vi "Main.vi"() -> ()   [LabVIEW 2020] (continued)
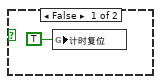
[diagram p2: hidden frame]
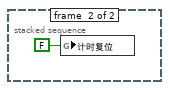
[diagram p3: hidden frame]
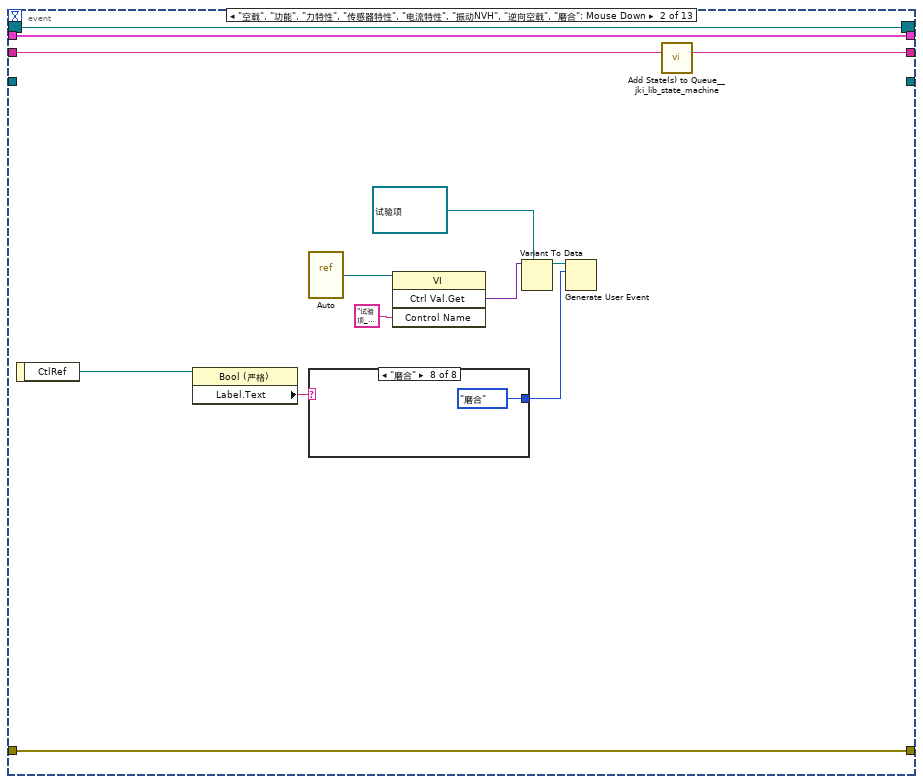
[diagram p4: hidden frame]
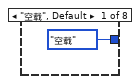
[diagram p5: hidden frame]
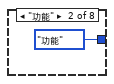
[diagram p6: hidden frame]
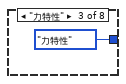
[diagram p7: hidden frame]
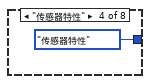
[diagram p8: hidden frame]
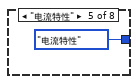
[diagram p9: hidden frame]
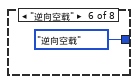
[diagram p10: hidden frame]
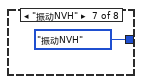
[diagram p11: hidden frame]
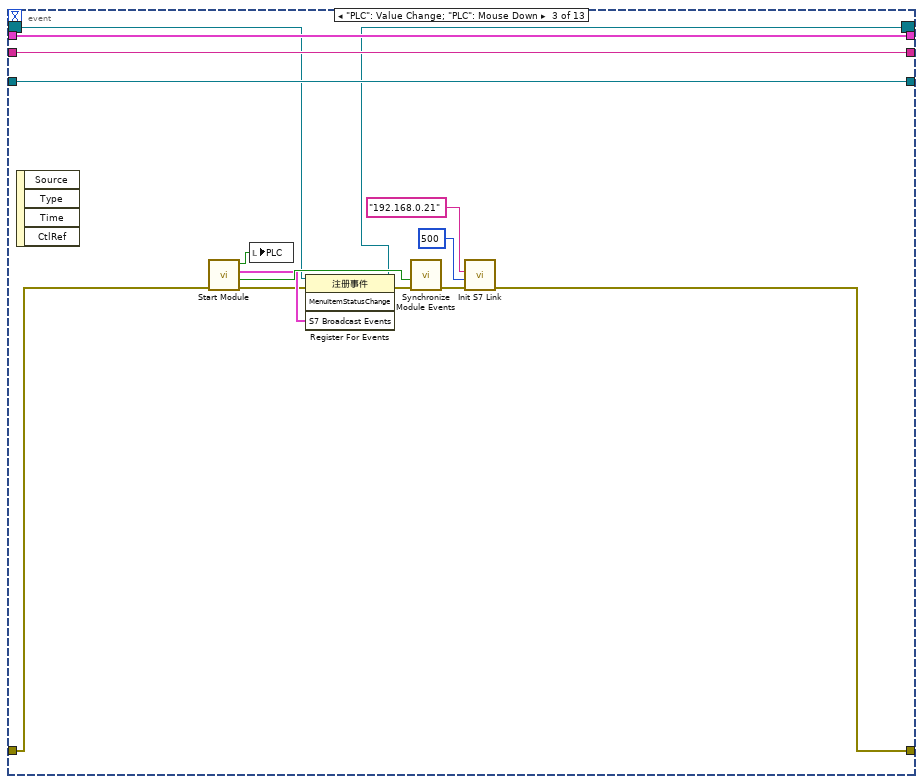
[diagram p12: hidden frame]
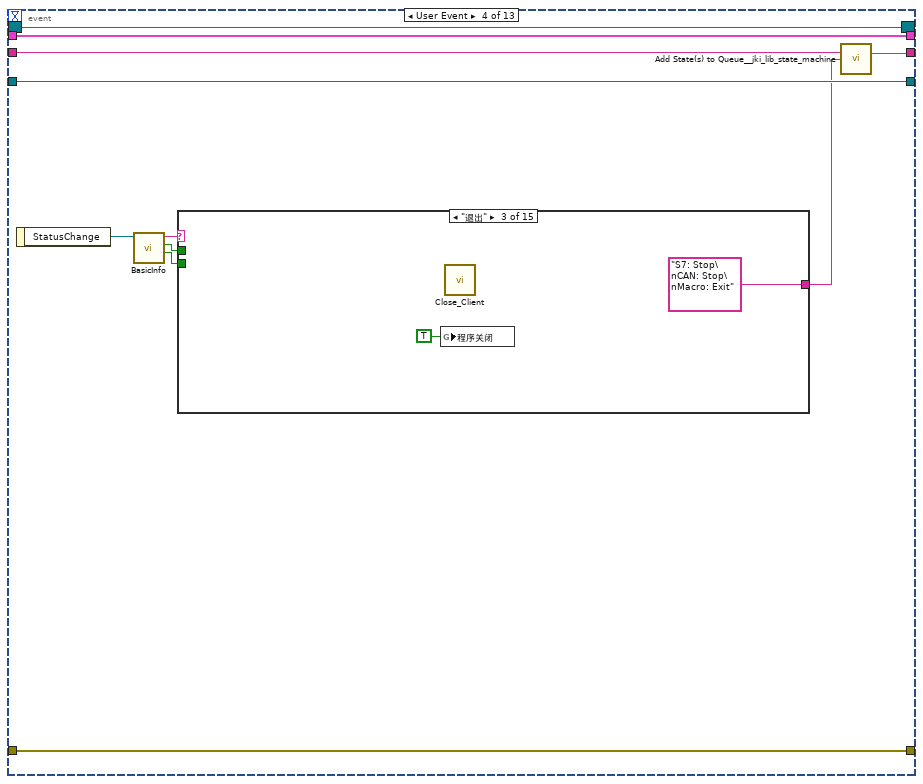
[diagram p13: hidden frame]
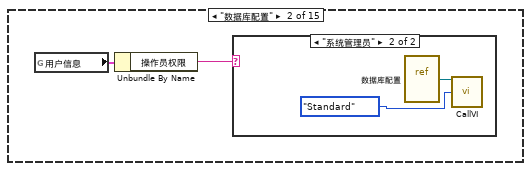
[diagram p15: hidden frame]
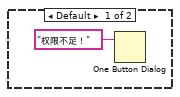
[diagram p16: hidden frame]
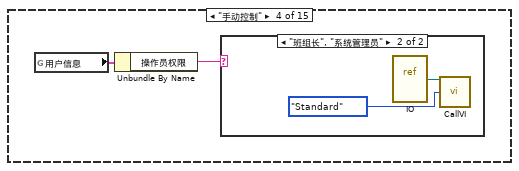
[diagram p17: hidden frame]
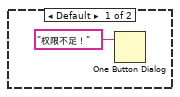
[diagram p18: hidden frame]
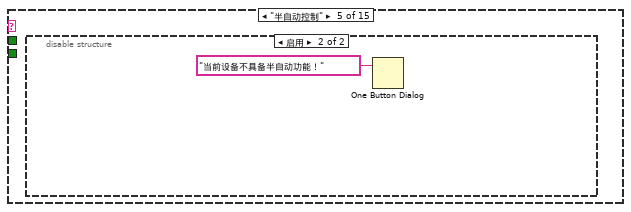
[diagram p19: hidden frame]
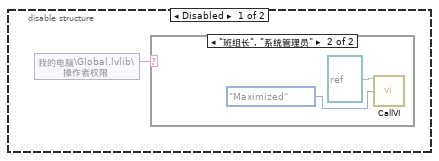
[diagram p20: hidden frame]
                n119 = case shown="真" w200 {
                  frame False {
                  }
                  frame True {
                    n120 = vi-ref "Auto.vi"() -> (w204:refnum<vi>)
                    n121 = invoke class="VI" method="Ctrl Val.Set"(reference=w204, "Control Name"="STEP" ("控件名"), "Value"="退出自动" ("控件名")) -> ()  [unwired: 2 in, 5 out]
                  }
                }
              }
            }
            n122 = call <vilib>:"Add State(s) to Queue__jki_lib_state_machine.vi"("State(s) in (\"\")"=w191) -> ("States Out"=w192:string)  [unwired: 14 in]
          }
          event "错误": Mouse Down {
            n123 = event-data() -> ()  [unwired: 1 in, 8 out]
            n124 = vi-ref "报警信息.vi"() -> (w207:refnum<vi>)
            n125 = call "CallVI.vi"("VI引用"=w207, "状态"=T3."Standard") -> ()  [unwired: 12 in, 2 out]
            n126 = call <vilib>:"Add State(s) to Queue__jki_lib_state_machine.vi"("State(s) in (\"\")"=w209) -> ("States Out"=w210:string)  [unwired: 14 in]
          }
          event Panel Close? {
            n127 = event-data() -> ()  [unwired: 1 in, 1 out]
            n128 = call "Close.vi"() -> ()  [unwired: 11 in, 1 out]
            n129 = global write "Global.vi" "程序关闭"(TRUE ("程序关闭")) -> ()
            n130 = call <vilib>:"Add State(s) to Queue__jki_lib_state_machine.vi"("State(s) in Front (\"\")"="S7: Stop\nMacro: Exit", "State(s) in (\"\")"=w219) -> ("States Out"=w218:string)  [unwired: 13 in]
            n131 = event-data("Discard?"=TRUE) -> ()  [unwired: 1 in, 1 out]
          }
          event "更换产品": Value Change {
            n132 = event-data() -> ("NewVal"=w222:refnum<vi>)  [unwired: 1 in, 5 out]
            n133 = stacked-sequence {
              tunnel: w222 -> [w228]
              tunnel: [w227] -> w220
              frame #0 {
                n134 = stacked-sequence {
                  tunnel: w228 -> [w236 _ _]
                  tunnel: [_ w239 _] -> w227
                  frame #0 {
                    n135 = disable-structure shown="禁用" {
                      disable-tunnel: w236 -> [w238 _]
                      frame Disabled {
                        n136 = control-ref of="子面板"() -> (w237:refnum<vi>)
                        n137 = call "Call_SubPanal.vi"("VI引用句柄"=w238, "SubPnl引用句柄"=w237) -> ()  [unwired: 9 in, 1 out]
                      }
                      frame Enabled {
                      }
                    }
                    n138 = vi-ref "Auto.vi"() -> (w235:refnum<vi>)
                    n139 = invoke class="VI" method="Ctrl Val.Get"(reference=w235, "Control Name"="产品变更_Event" ("控件名")) -> ("Get Control Value Variant"=w233:variant)  [unwired: 2 in, 3 out]
                    n140 = global read "Global.vi" "产品型号"() -> (w230:string)
                    n141 = Variant To Data(type=refnum<user-event> refnum ("产品变更_Event"), Variant=w233) -> (data=w231:refnum<user-event>, error out=w229:errorcluster)  [unwired: 1 in]
                    n142 = Generate User Event(user event=w231, event data cluster=w230, error in=w229) -> ()  [unwired: 1 in, 2 out]
                    n143 = local write "产品型号"(w230) -> ()
                  }
                  frame #1 {
                    n144 = global read "Global.vi" "启用CAN"() -> (w240:bool)
                    n145 = case shown="真" w240 {
                      tunnel: ["CAN: Stop" "CAN: Stop\nIdle\nCAN: Start"] -> w239
                      frame False {
                      }
                      frame True {
                      }
                    }
                  }
                  frame #2 {
                    n146 = control-ref of="磨合"() -> (w243:refnum<vi>)
                    n147 = control-ref of="空载"() -> (w248:refnum<vi>)
                    n148 = control-ref of="功能"() -> (w249:refnum<vi>)
                    n149 = control-ref of="力特性"() -> (w250:refnum<vi>)
                    n150 = control-ref of="电流特性"() -> (w247:refnum<vi>)
                    n151 = control-ref of="传感器特性"() -> (w246:refnum<vi>)
                    n152 = control-ref of="逆向空载"() -> (w245:refnum<vi>)
                    n153 = control-ref of="振动NVH"() -> (w244:refnum<vi>)
                    n154 = global read "Global.vi" "试验项目"() -> (w253:bool[])
                    n155 = Build Array(w248, w249, w250, w247, w246, w245, w244, w243) -> (w252:refnum<vi>[])
                    n156 = for {
                      tunnel: w252 -> [w257] mode=indexing
                      tunnel: w253 -> [w258] mode=indexing
                      shift-right: [w254] -> _
                      shift-left: 2095 -> [w255]
                      i -> [w256]
                      n157 = case shown="真" w258 {
                        tunnel: w257 -> [w259 w267]
                        tunnel: w256 -> [_ _]
                        tunnel: w255 -> [w261 w264]
                        tunnel: [w261 w262] -> w254
                        frame False {
                          n158 = property class="Bool (严格)"(reference=w259, "Top"=2000) -> ()  [unwired: 1 in, 2 out]
                        }
                        frame True {
                          n159 = Add(x=w264, y=115) -> (x+y=w262:i32)
                          n160 = Bundle(w262, 1300) -> (w265:cluster{i32, i32})  [unwired: 1 in]
                          n161 = property class="Bool (严格)"(reference=w267, "Position"=w265) -> ()  [unwired: 1 in, 2 out]
                        }
                      }
                    }
                  }
                }
              }
            }
            n162 = call <vilib>:"Add State(s) to Queue__jki_lib_state_machine.vi"("State(s) in Front (\"\")"=w220, "State(s) in (\"\")"=w223) -> ("States Out"=w224:string)  [unwired: 13 in]
          }
          event "Andon": Value Change {
            n163 = event-data() -> ("NewVal"=w272:enum32{"未选择", "缺料报警", "质量报警", "故障报警"})  [unwired: 1 in]
            n164 = case shown="\"未选择\", 默认" w272 {
              tunnel: [enum16{"设备离线", "设备正常", "设备缺料", "设备故障", "质量报警"}."设备正常" ("设备状态") enum16{"设备离线", "设备正常", "设备缺料", "设备故障", "质量报警"}."设备缺料" ("设备状态") enum16{"设备离线", "设备正常", "设备缺料", "设备故障", "质量报警"}."质量报警" ("设备状态") enum16{"设备离线", "设备正常", "设备缺料", "设备故障", "质量报警"}."设备故障" ("设备状态")] -> w270
              frame "未选择", Default {
              }
              frame "缺料报警" {
              }
              frame "质量报警" {
              }
              frame "故障报警" {
              }
            }
            n165 = local read "userName"() -> (w269:string)
            n166 = Bundle By Name(cluster=T4 {"设备名称"="最终性能试验台1", "操作人员"="", "设备状态"=enum."设备离线", "附加信息"=""} ("设备信息"), "操作人员"=w269, "设备状态"=w270) -> (w268:T4)
            n167 = call "Change_Client.vi"("设备信息"=w268) -> ()  [unwired: 10 in, 1 out]
          }
        }
      }
      frame "---------- Core ----------" {
        n168 = call <vilib>:"Add State(s) to Queue__jki_lib_state_machine.vi"("State(s) in (\"\")"=w286) -> ("States Out"=w285:string)  [unwired: 14 in]
      }
      frame Default {
        w298 = 42 items=["No error", "Argument error", "Memory is full", "Out of zone", "End of file", "File already open", "Generic file I/O error", "File not found", "File permission error", "Disk is full", "Duplicate path", "Too many files open", "System feature not enabled", "Resource file not found", "Cannot add resource", "Resource not found", "Image not found", "Image memory error", "Pen does not exist", "Config type invalid", "Config token not found", "Config parse error", "Config memory error", "Bad external code format", "Bad external code offset", "External code not present", "Null window", "Destroy window error", "Null menu", "Print aborted", "Bad print record", "Print driver error", "Windows error during printing", "Memory error during printing", "Print dialog error", "Generic print error", "Invalid device refnum", "Device not found", "Device parameter error", "Device unit error", "Cannot open device", "Device call aborted", "Generic error", "Cancelled by user", "Object ID too low", "Object ID too high", "Object not in heap", "Unknown heap", "Unknown object (invalid DefProc)", "Unknown object (DefProc not in table)", "Message out of range", "Invalid (null) method", "Unknown message", "Manager call not supported", "Bad address", "Network operation in progress", "Network operation timed out", "Connection is busy", "Network attribute not supported", "Network error", "Address in use", "System out of memory", "Connection aborted", "Connection refused", "Not connected", "Already connected", "Connection closed", "Initialization error (interapplication manager)", "Bad occurrence", "Wait on unbound occurrence handler", "Occurrence queue overflow", "Datalog type conflict", "Unused", "Unrecognized type (interapplication manager)", "Memory corrupt", "Failed to make temporary DLL", "Old CIN version", "Drag socket not found", "Failed to load drop-object", "Failed to register OLE object", "Failed to release OLE object", "Format specifier type mismatch", "Unknown format specifier", "Too few format specifiers", "Too many format specifiers", "Scan failed", "Newer CIN version", "Error converting to variant", "Runtime menu error", "Password tampered", "Variant attribute not found", "Incompatible variant data type", "Event data is not available", "Event Store is not present", "Occurrence is not found", "Event Queue is not created", "Event info is not available", "Refnum passed is NULL", "Error retrieving Class GUID", "Error retrieving CoClass GUID", "Error retrieving TypeLib GUID.", "Bad built application magic bytes.", "Specific driver is different from the specific driver associated with the Logical Name.", "There is no session opened to the class driver.", "Max Error", "MAX - Error with config objects", "MAX - Error loading configuration", "MAX - Group not supported"]
        # "Current State"
        n169 = Format Into String(format string="Software Exception: Unhandled State \"%s\"." ("message"), error in=w294, w289) -> (resulting string=w297:string, error out=w296:errorcluster)  [unwired: 1 in]
        n170 = call <vilib>:"Error Cluster From Error Code.vi"("show call chain? (False)"=TRUE, "error in (no error)"=w296, "error message (\"\")"=w297, "error code (0)"=w298) -> ("error out"=w295:errorcluster)  [unwired: 5 in]
        n171 = call <vilib>:"Add State(s) to Queue__jki_lib_state_machine.vi"("State(s) in (\"\")"=w293) -> ("States Out"=w292:string)  [unwired: 14 in]
      }
      frame "Initialize Core Data" {
        # "originally closed?"
        # "exe?"
        n172 = property class="VI"() -> ("Front Panel.Open"=w309:bool)  [unwired: 2 in, 2 out]
        n173 = property class="App"() -> ("App.Kind"=w308:T5)  [unwired: 2 in, 2 out]
        n174 = control-ref of="Current VI Reference"() -> (w302:refnum<vi>)
        n175 = Not(x=w309) -> (.not. x?=w306:bool)
        n176 = Equal?(x=w308, y=T5."Run Time System" ("Application:Kind")) -> (x = y?=w305:bool)
        n177 = Or(x=w306, y=w305) -> (x .or. y?=w303:bool)
        n178 = Bundle By Name(cluster=w304, "Core.Current VI Reference"=w302, "Core.Close Panel on Exit?"=w303) -> (w311:T7)
        n179 = call <vilib>:"Add State(s) to Queue__jki_lib_state_machine.vi"("State(s) in (\"\")"=w313) -> ("States Out"=w312:string)  [unwired: 14 in]
      }
      frame "Error Handler" {
        n180 = call <vilib>:"General Error Handler.vi"("error in (no error)"=w317) -> ()  [unwired: 10 in, 5 out]
        n181 = call <vilib>:"Add State(s) to Queue__jki_lib_state_machine.vi"("State(s) in Front (\"\")"="/* Post Error States", "State(s) in (\"\")"=w321) -> ("States Out"=w320:string)  [unwired: 13 in]
      }
      frame "Exit" {
        n182 = call <vilib>:"Add State(s) to Queue__jki_lib_state_machine.vi"("State(s) in (\"\")"=w328) -> ("States Out"=w327:string)  [unwired: 14 in]
        n183 = Quit LabVIEW() -> ()  [unwired: 1 in]
      }
      frame "--------- Library --------" {
        n184 = call <vilib>:"Add State(s) to Queue__jki_lib_state_machine.vi"("State(s) in (\"\")"=w334) -> ("States Out"=w333:string)  [unwired: 14 in]
      }
      frame "S7: Initialize" {
        n185 = property on="PLC" class="Bool (严格)"("Val(Sgnl)"=FALSE ("值(信号)")) -> ()  [unwired: 2 in, 2 out]
      }
      frame "S7: Stop" {
        n186 = call "Stop Module.vi"("error in (no error)"=w343) -> ("error out"=w342:errorcluster)  [unwired: 10 in]
        n187 = call <vilib>:"Add State(s) to Queue__jki_lib_state_machine.vi"("State(s) in (\"\")"=w344) -> ("States Out"=w345:string)  [unwired: 14 in]
      }
      frame "CAN: Start" {
        n188 = while {
          stop <- w356 stop-if-true
          n189 = vi-ref "CAN.vi"() -> (w359:refnum<vi>)
          n190 = call "CallVI.vi"("VI引用"=w359, "状态"=T3."Hidden") -> ("VI引用OUT"=w355:refnum<vi>, "错误输出"=w357:errorcluster)  [unwired: 12 in]
          n191 = property class="VI"(reference=w355, error in=w357) -> ("Exec.State"=w358:T8)  [unwired: 2 out]
          n192 = case shown="\"Run top level\"" w358 {
            tunnel: [w360 TRUE TRUE] -> w356
            frame "Bad", Default {
              n193 = Two Button Dialog(message="CAN卡打开失败！" ("消息"), 1:"重试" ("F按钮名称（“取消”）"), 2:"忽略" ("T按钮名称（“确定”）")) -> (T button?=w360:bool)
            }
            frame "Run top level" {
            }
            frame "Running" {
            }
          }
        }
        n194 = call <vilib>:"Add State(s) to Queue__jki_lib_state_machine.vi"("State(s) in (\"\")"=w350) -> ("States Out"=w351:string)  [unwired: 14 in]
      }
      frame "CAN: Stop" {
        n195 = vi-ref "CAN.vi"() -> (w368:refnum<vi>)
        n196 = invoke class="VI" method="Ctrl Val.Set"(reference=w368, "Control Name"="Stop" ("控件名"), "Value"=TRUE) -> ()  [unwired: 2 in, 5 out]
        n197 = call <vilib>:"Add State(s) to Queue__jki_lib_state_machine.vi"("State(s) in (\"\")"=w371) -> ("States Out"=w372:string)  [unwired: 14 in]
      }
      frame "---------- Data ----------" {
        n198 = call <vilib>:"Add State(s) to Queue__jki_lib_state_machine.vi"("State(s) in (\"\")"=w380) -> ("States Out"=w379:string)  [unwired: 14 in]
      }
      frame "Data: Initialize" {
        w385 = T9 {"Current VI Reference"=refnum, "Close Panel on Exit?"=FALSE}  # Core
        w387 = TRUE  # Your Boolean data
        w386 = ""  # Your string data
        n199 = global write "Global.vi" "程序关闭"(FALSE ("程序关闭")) -> ()
        n200 = global write "Global.vi" "计时开始"(FALSE ("计时结束")) -> ()
        n201 = Bundle("Core"=w385, "Your Boolean data"=w387, "Your string data"=w386) -> (w389:T7)  [unwired: 1 in]
        n202 = call <vilib>:"Add State(s) to Queue__jki_lib_state_machine.vi"("State(s) in (\"\")"=w391) -> ("States Out"=w390:string)  [unwired: 14 in]
      }
      frame "Data: Cleanup" {
        n203 = Unbundle By Name(w394) -> ("Core.Current VI Reference"=w397:refnum<vi>)
        n204 = Close Reference(reference=w397, error in (no error)=w396) -> (error out=w395:errorcluster)
        n205 = call <vilib>:"Add State(s) to Queue__jki_lib_state_machine.vi"("State(s) in (\"\")"=w399) -> ("States Out"=w398:string)  [unwired: 14 in]
      }
      frame "---------- UI ----------" {
        # "Do not put any code in this frame.\n(It is a separator no-op. You can make a copy of this frame to create a new UI frame)"
        n206 = call <vilib>:"Add State(s) to Queue__jki_lib_state_machine.vi"("State(s) in (\"\")"=w405) -> ("States Out"=w404:string)  [unwired: 14 in]
      }
      frame "UI: Initialize" {
        n207 = disable-structure shown="启用" {
          disable-tunnel: [w415 _] -> w409
          disable-tunnel: w406 -> [w413 _]
          frame Enabled {
            n208 = vi-ref "Auto.vi"() -> (w414:refnum<vi>)
            n209 = invoke on="子面板" class="SubPnl" method="Insert VI"(error in=w413, "VI Ref"=w414) -> (error out=w418:errorcluster)  [unwired: 2 in, 3 out]
            n210 = invoke class="VI" method="Run VI"(reference=w414, error in=w418, "Wait until done"=FALSE ("结束前等待"), "Auto Dispose Ref"=TRUE ("自动销毁引用")) -> (error out=w415:errorcluster)  [unwired: 1 in, 4 out]
          }
          frame Disabled {
            n211 = vi-ref "Auto.vi"() -> (w420:refnum<vi>)
            n212 = call "CallVI.vi"("VI引用"=w420, "状态"=T3."Maximized") -> ()  [unwired: 12 in, 2 out]
          }
        }
        n213 = call <vilib>:"Add State(s) to Queue__jki_lib_state_machine.vi"("State(s) in (\"\")"=w412) -> ("States Out"=w411:string)  [unwired: 14 in]
      }
      frame "UI: Init" {
        n214 = stacked-sequence {
          tunnel: w422 -> [_ _ _ _ _]
          frame #0 {
            n215 = call "Open.vi"() -> ()  [unwired: 11 in, 1 out]
          }
          frame #1 {
            n216 = global write "Global.vi" "程序关闭"(FALSE ("程序关闭")) -> ()
            n217 = control-ref of="电流特性"() -> (w431:refnum<vi>)
            n218 = control-ref of="空载"() -> (w434:refnum<vi>)
            n219 = control-ref of="力特性"() -> (w432:refnum<vi>)
            n220 = control-ref of="功能"() -> (w433:refnum<vi>)
            n221 = global write "A180648.vi" "LED-电流特性"(w431) -> ()
            n222 = global write "A180648.vi" "LED-空载"(w434) -> ()
            n223 = global write "A180648.vi" "LED-力特性"(w432) -> ()
            n224 = global write "A180648.vi" "LED-功能"(w433) -> ()
            n225 = control-ref of="逆向空载"() -> (w430:refnum<vi>)
            n226 = control-ref of="振动NVH"() -> (w428:refnum<vi>)
            n227 = control-ref of="传感器特性"() -> (w429:refnum<vi>)
            n228 = control-ref of="磨合"() -> (w427:refnum<vi>)
            n229 = global write "A180648.vi" "LED-传感器特性"(w429) -> ()
            n230 = global write "A180648.vi" "LED-逆向空载"(w430) -> ()
            n231 = global write "A180648.vi" "LED-振动NVH"(w428) -> ()
            n232 = global write "A180648.vi" "LED-磨合"(w427) -> ()
          }
          frame #2 {
            w442 = 0
            n233 = shared-variable "我的电脑\\Global.lvlib\\总成追溯码"("   " ("工位追溯码")) -> ()  [unwired: 1 in, 1 out]
            n234 = global write "Global.vi" "生产数量"(w442) -> ()
            n235 = global write "Global.vi" "合格数量"(w442) -> ()
            n236 = global read "Global.vi" "用户信息"() -> (w439:T10)
            n237 = global read "Global.vi" "联机模式"() -> (w436:enum16{"单机", "追溯"})
            n238 = Unbundle By Name(w439) -> ("用户名"=→"userName":string, "用户权限"=→"userStatus":string)
            n239 = case shown="\"追溯\"" w436 {
              tunnel: ["联网" ("connectionMode") "单机" ("connectionMode")] -> w443
              frame "追溯" {
              }
              frame "单机", Default {
              }
            }
            "connectionMode" <- w443
            "产品型号" <- "" ("产品型号")
          }
          frame #3 {
            n240 = control-ref of="提示信息"() -> (w447:refnum<vi>)
            n241 = control-ref of="自动"() -> (w448:refnum<vi>)
            n242 = control-ref of="错误"() -> (w449:refnum<vi>)
            n243 = control-ref of="Result"() -> (w450:refnum<vi>)
            n244 = control-ref of="更换产品"() -> (w446:refnum<vi>)
            n245 = global write "Global.vi" "提示信息"(w447) -> ()
            n246 = global write "Global.vi" "程序自动"(w448) -> ()
            n247 = global write "Global.vi" "报警图标"(w449) -> ()
            n248 = global write "Global.vi" "Result"(w450) -> ()
            n249 = global write "Global.vi" "更换产品"(w446) -> ()
          }
          frame #4 {
            n250 = global read "Global.vi" "Result"() -> (w453:refnum<vi>)
            n251 = property class="Tbl"(reference=w453, "Row Headers[]"=string[] [], "Value"=string[][] []) -> ()  [unwired: 1 in, 2 out]
            n252 = call "Start_Client.vi"() -> ()  [unwired: 12 in]
          }
        }
        n253 = call <vilib>:"Add State(s) to Queue__jki_lib_state_machine.vi"("State(s) in (\"\")"=w426) -> ("States Out"=w425:string)  [unwired: 14 in]
      }
      frame "UI: Config" {
        n254 = vi-ref "Config.vi"() -> (w456:refnum<vi>)
        n255 = call "CallVI.vi"("VI引用"=w456, "状态"=T3."Standard") -> ()  [unwired: 12 in, 2 out]
        n256 = call <vilib>:"Add State(s) to Queue__jki_lib_state_machine.vi"("State(s) in (\"\")"=w461) -> ("States Out"=w460:string)  [unwired: 14 in]
      }
      frame "UI: Cursor Set" {
        # "Argument"
        n257 = case shown="\"Idle\", 默认" w464 {
          tunnel: w466 -> [w471 w473]
          tunnel: [w470 w472] -> w465
          frame "Idle", Default {
            n258 = call <vilib>:"Unset Busy.vi"("error in (no error)"=w471) -> ("error out"=w470:errorcluster)  [unwired: 10 in]
          }
          frame "Busy" {
            n259 = call <vilib>:"Set Busy.vi"("error in (no error)"=w473) -> ("error out"=w472:errorcluster)  [unwired: 9 in, 1 out]
          }
        }
        n260 = call <vilib>:"Add State(s) to Queue__jki_lib_state_machine.vi"("State(s) in (\"\")"=w469) -> ("States Out"=w468:string)  [unwired: 14 in]
      }
      frame "UI: Front Panel State" {
        # "Argument"
        n261 = Unbundle By Name(w478) -> ("Core.Current VI Reference"=w477:refnum<vi>)
        n262 = case shown="\"Close\"" w476 {
          tunnel: w480 -> [w486 w499]
          tunnel: [w488 w500] -> w479
          tunnel: w477 -> [w487 w497]
          frame "Open", Default {
            n263 = property class="VI"(reference=w487, error in=w486) -> (reference out=w484:refnum<vi>, error out=w485:errorcluster, "Front Panel.Open"=w483:bool)
            n264 = case shown="假" w483 {
              tunnel: [w491 w494] -> w488
              tunnel: w485 -> [w490 w494]
              tunnel: w484 -> [w489 _]
              frame False {
                n265 = invoke class="VI" method="FP.Open"(reference=w489, error in=w490, "Activate"=TRUE, "State"=T3."Standard") -> (error out=w491:errorcluster)  [unwired: 1 in, 4 out]
              }
              frame True {
              }
            }
          }
          frame "Close" {
            n266 = property class="VI"(reference=w497, error in=w499) -> (reference out=w496:refnum<vi>, error out=w498:errorcluster, "Front Panel.Open"=w495:bool)
            n267 = case shown="真" w495 {
              tunnel: [w501 w504] -> w500
              tunnel: w498 -> [w501 w503]
              tunnel: w496 -> [_ w502]
              frame False {
              }
              frame True {
                n268 = invoke class="VI" method="FP.Close"(reference=w502, error in=w503) -> (error out=w504:errorcluster)  [unwired: 1 in, 2 out]
              }
            }
          }
        }
        n269 = call <vilib>:"Add State(s) to Queue__jki_lib_state_machine.vi"("State(s) in (\"\")"=w482) -> ("States Out"=w481:string)  [unwired: 14 in]
      }
      frame "---------- Macro ----------" {
        n270 = call <vilib>:"Add State(s) to Queue__jki_lib_state_machine.vi"("State(s) in (\"\")"=w510) -> ("States Out"=w509:string)  [unwired: 14 in]
      }
      frame "Macro: Initialize" {
        n271 = call <vilib>:"Add State(s) to Queue__jki_lib_state_machine.vi"("State(s) in Front (\"\")"="Data: Initialize\nInitialize Core Data\nS7: Initialize\nIdle\nUI: Init\nUI: Front Panel State >> Open\nUI: Initialize\nUI: Config", "State(s) in (\"\")"=w517) -> ("States Out"=w516:string)  [unwired: 13 in]
      }
      frame "Macro: Exit" {
        n272 = Unbundle By Name(w526) -> ("Core.Close Panel on Exit?"=w525:bool)
        n273 = Select(t="UI: Front Panel State >> Close", s=w525, f="") -> (s? t:f=w522:string)
        n274 = call <vilib>:"Add State(s) to Queue__jki_lib_state_machine.vi"("State(s) in (\"\")"=w522, "State(s) at Back (\"\")"="Data: Cleanup\nExit") -> ("States Out"=w520:string)  [unwired: 13 in]
        n275 = call <vilib>:"Add State(s) to Queue__jki_lib_state_machine.vi"("State(s) in Front (\"\")"=w520, "State(s) in (\"\")"=w529) -> ("States Out"=w528:string)  [unwired: 13 in]
      }
    }
  }
  n276 = call-dynamic "Cleanup.vi"("MenuStrip in"=w6) -> ()  [unwired: 10 in, 1 out]
